vi "ImageToSound.vi"() -> ()   [LabVIEW 2014]
uses:
  <vilib>/Analysis/2dsp.llb/Inverse Real FFT.vi
  <vilib>/Analysis/NI_AALPro.lvlib
panel:
  in  "Sound Output Selection":enum16{"Computer Speakers", "DAQ"}(ring)=enum."DAQ"
  out "Picture":picture
  in  "Path":path=path "U:/phys 434/Project/Suggested Images For Processing/OrlalaAndElana.JPG"
  in  "Sampling Rate":dbl=50000.0
  out "Waveform Graph 3":waveform(dbl)(graph)={"t0"=timestamp(0 s since 1904-01-01), "dt"=2e-05, "Y"=array[1227520 elements]}
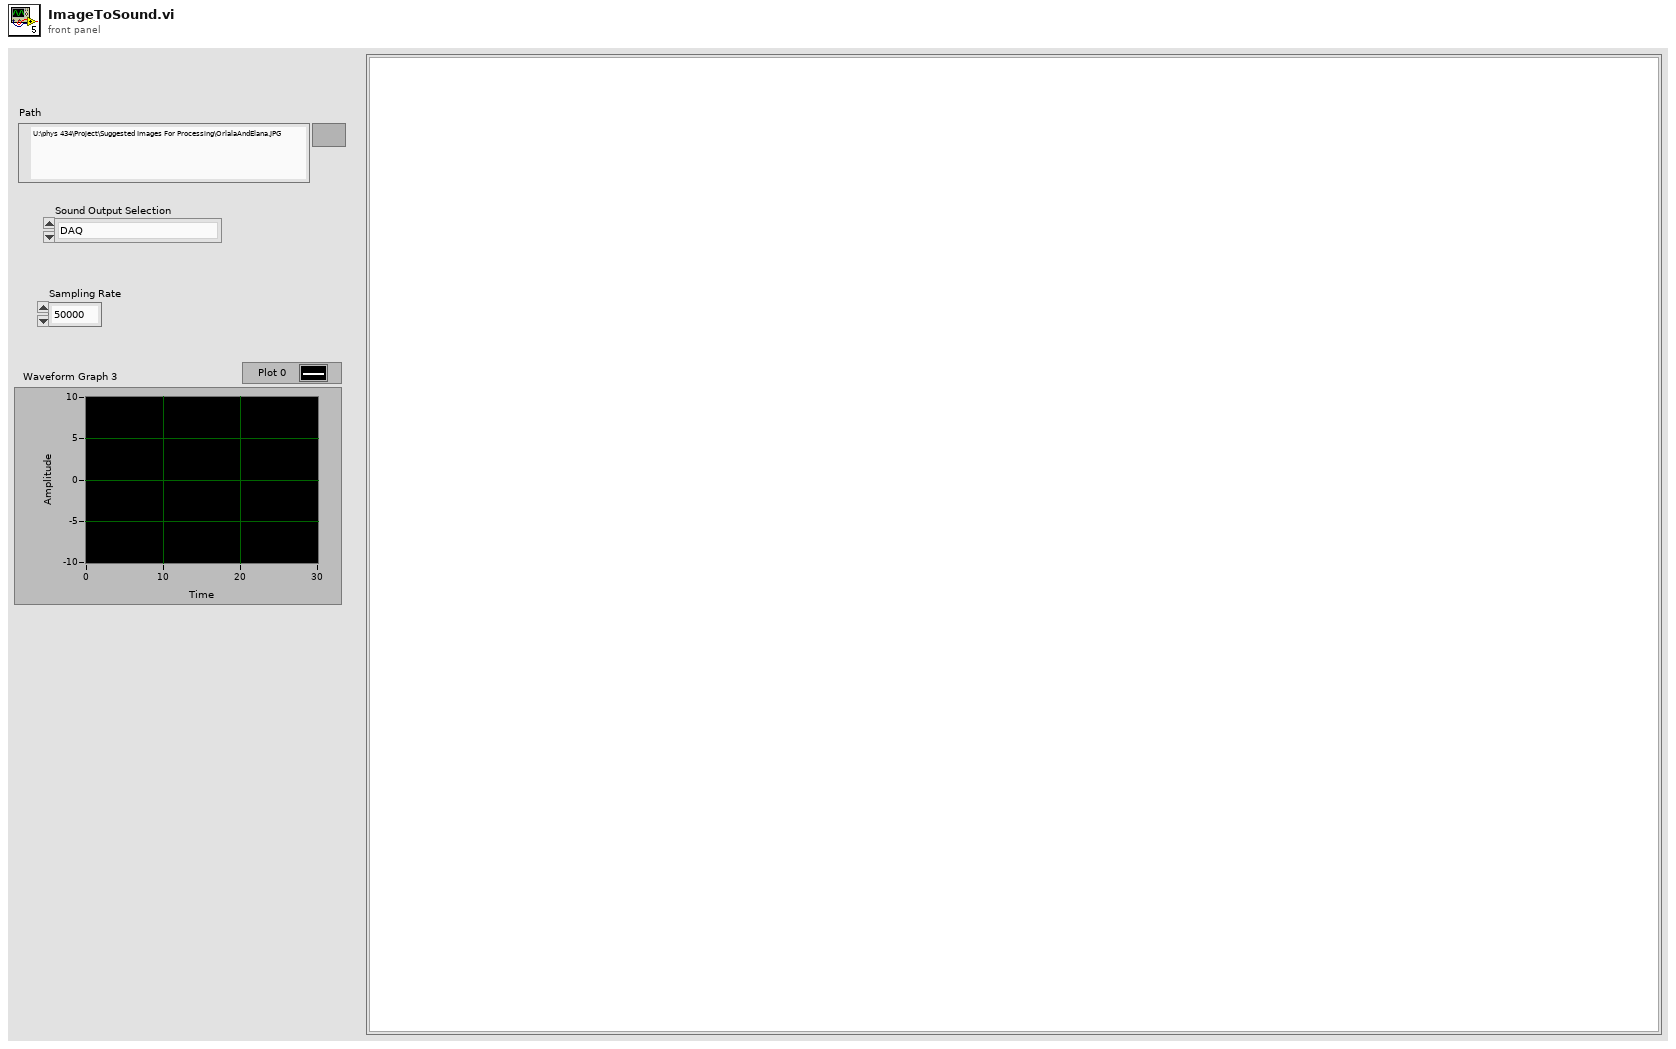
[diagram p1: front panel]
types:
  T1 = typedef "imagedata.ctl" = cluster{"image type":i32, "image depth":i32, "image":u8[], "mask":u8[], "colors":u32[], "Rectangle":cluster{"left":i16, "top":i16, "right":i16, "bottom":i16}}
  T2 = cluster{"left":i16, "top":i16, "right":i16, "bottom":i16}
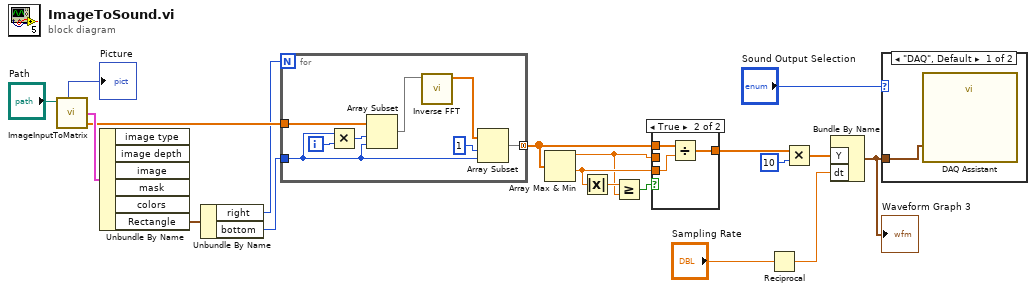
[diagram p0: block diagram]
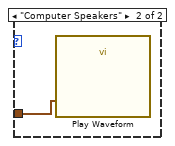
[diagram p2: hidden frame]
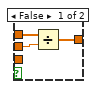
[diagram p3: hidden frame]
diagram:
  n1 = call "ImageInputToMatrix.vi"("Path"="Path") -> ("Picture"=→"Picture":picture, "image data"=w18:T1, "Image Data Vector"=w17:dbl[])  [unwired: 4 in, 1 out]
  n2 = Unbundle By Name(w18) -> ("Rectangle"=w19:T2)  [unwired: 5 out]
  n3 = Unbundle By Name(w19) -> ("right"=w16:i16, "bottom"=w15:i16)
  n4 = for {
    N: w16 -> [_]
    tunnel: w17 -> [w26]
    tunnel: w15 -> [w23]
    tunnel: [w20] -> w5 mode=concatenating
    i -> [w25]
    n5 = Multiply(x=w23, y=w25) -> (x*y=w27:i32)
    n6 = Array Subset(array=w26, index=w27, length=w23) -> (w22:dbl[])
    n7 = call-poly <vilib>:"Inverse FFT.vi"("FFT {X}"=w22) -> ("X"=w21:dbl[])  [unwired: 9 in, 1 out]
    n8 = Array Subset(array=w21, index=1, length=w23) -> (w20:dbl[])
  }
  n9 = Array Max & Min(array=w5) -> (max value=w6:dbl, min value=w9:dbl)  [unwired: 2 out]
  n10 = Absolute Value(x=w9) -> (abs(x)=w10:dbl)
  n11 = Greater Or Equal?(x=w10, y=w6) -> (x >= y?=w7:bool)
  n12 = case shown="True" w7 {
    tunnel: w9 -> [_ w33]
    tunnel: [w29 w32] -> w8
    tunnel: w6 -> [w30 _]
    tunnel: w5 -> [w28 w31]
    frame False {
      n13 = Divide(x=w28, y=w30) -> (x/y=w29:dbl[])
    }
    frame True {
      n14 = Divide(x=w31, y=w33) -> (x/y=w32:dbl[])
    }
  }
  n15 = Reciprocal(x="Sampling Rate") -> (1/x=w12:dbl)
  n16 = Multiply(x=w8, y=10) -> (x*y=w4:dbl[])
  n17 = Bundle By Name("Y"=w4, "dt"=w12) -> (w3:waveform(dbl))  [unwired: 1 in]
  "Waveform Graph 3" <- w3
  n18 = case shown="\"DAQ\", Default" "Sound Output Selection" {
    tunnel: w3 -> [w34 w35]
    frame "DAQ", Default {
      n19 = call "DAQ Assistant"("data"=w34) -> ()  [unwired: 17 in, 2 out]
    }
    frame "Computer Speakers" {
      n20 = call "Play Waveform"("Data"=w35) -> ()  [unwired: 18 in, 1 out]
    }
  }
